vi "FlexMag - 23-03-2023.vi"() -> ()   [LabVIEW 2018] (continued)
              }
              frame #16 {
                n12360 = local read "ch4-3 transfer"() -> (w17570:bool)
                n12361 = case shown="True" w17570 {
                  frame False {
                  }
                  frame True {
                    n12362 = local read "ABORT"() -> (w17571:bool)
                    n12363 = case shown="False" w17571 {
                      frame False {
                        n12364 = local write "trns 4-3 led 7"(TRUE ("trns 1-2 led 1")) -> ()
                        n12365 = Wait (ms)(milliseconds to wait=u32 100) -> ()  [unwired: 1 out]
                      }
                      frame True {
                      }
                    }
                  }
                }
              }
              frame #17 {
                n12366 = local read "ch4-3 transfer"() -> (w17574:bool)
                n12367 = case shown="True" w17574 {
                  frame False {
                  }
                  frame True {
                    n12368 = local read "ABORT"() -> (w17575:bool)
                    n12369 = case shown="False" w17575 {
                      frame False {
                        n12370 = disable-structure shown="Enabled" {
                          frame Disabled {
                            n12371 = while {
                              i -> [w17580]
                              stop <- w17581 stop-if-true
                              n12372 = Greater Or Equal?(x=w17580, y=100) -> (x >= y?=w17578:bool)
                              n12373 = case shown="True" w17578 {
                                frame False {
                                }
                                frame True {
                                n12374 = local write "Warning Message"("Transfer process canceled!\nRight Slow Sensor problem" ("Warning Message")) -> ()
                                n12375 = local write "trns error"(TRUE ("TRNS error")) -> ()
                                }
                              }
                              n12376 = local read "Cnt_Right_Slow DI"() -> (w17576:bool)
                              n12377 = case shown="True" w17576 {
                                tunnel: [TRUE ("CH1_Trns_BP_Left_DO") FALSE ("CH1_Trns_BP_Left_DO")] -> w17577
                                frame False {
                                }
                                frame True {
                                n12378 = Wait Until Next ms Multiple(millisecond multiple=u32 200) -> ()  [unwired: 1 out]
                                n12379 = local write "Cnt_Right_Slow DO"(FALSE ("CH1_Trns_BP_Left_DO")) -> ()
                                }
                              }
                              n12380 = local read "ch4-3 transfer"() -> (w17584:bool)
                              n12381 = local read "ABORT"() -> (w17583:bool)
                              n12382 = Not(x=w17584) -> (.not. x?=w17582:bool)
                              n12383 = Compound Arithmetic op=OR(w17577, w17583, w17582) -> (w17581:bool)
                            }
                          }
                          frame Enabled {
                          }
                        }
                      }
                      frame True {
                      }
                    }
                  }
                }
              }
              frame #18 {
                n12384 = local read "ch4-3 transfer"() -> (w17591:bool)
                n12385 = case shown="True" w17591 {
                  frame False {
                  }
                  frame True {
                    n12386 = local read "ABORT"() -> (w17592:bool)
                    n12387 = case shown="False" w17592 {
                      frame False {
                        n12388 = local write "trns 4-3 led 8"(TRUE ("trns 1-2 led 1")) -> ()
                        n12389 = Wait (ms)(milliseconds to wait=u32 100) -> ()  [unwired: 1 out]
                      }
                      frame True {
                      }
                    }
                  }
                }
              }
              frame #19 {
                n12390 = local read "ch4-3 transfer"() -> (w17595:bool)
                n12391 = case shown="True" w17595 {
                  frame False {
                  }
                  frame True {
                    n12392 = local read "ABORT"() -> (w17596:bool)
                    n12393 = case shown="False" w17596 {
                      frame False {
                        n12394 = disable-structure shown="Enabled" {
                          frame Disabled {
                            n12395 = while {
                              i -> [w17601]
                              stop <- w17602 stop-if-true
                              n12396 = Greater Or Equal?(x=w17601, y=100) -> (x >= y?=w17599:bool)
                              n12397 = case shown="True" w17599 {
                                frame False {
                                }
                                frame True {
                                n12398 = local write "Warning Message"("Transfer process canceled!\nRight Limit Sensor problem" ("Warning Message")) -> ()
                                n12399 = local write "trns error"(TRUE ("TRNS error")) -> ()
                                }
                              }
                              n12400 = local read "Cnt_Right_Limit DI"() -> (w17597:bool)
                              n12401 = case shown="True" w17597 {
                                tunnel: [TRUE ("CH1_Trns_BP_Left_DO") FALSE ("CH1_Trns_BP_Left_DO")] -> w17598
                                frame False {
                                }
                                frame True {
                                n12402 = Wait Until Next ms Multiple(millisecond multiple=u32 200) -> ()  [unwired: 1 out]
                                n12403 = local write "Cnt_Right_Limit DO"(FALSE ("CH1_Trns_BP_Left_DO")) -> ()
                                }
                              }
                              n12404 = local read "ch4-3 transfer"() -> (w17605:bool)
                              n12405 = local read "ABORT"() -> (w17604:bool)
                              n12406 = Not(x=w17605) -> (.not. x?=w17603:bool)
                              n12407 = Compound Arithmetic op=OR(w17598, w17604, w17603) -> (w17602:bool)
                            }
                          }
                          frame Enabled {
                            w17613 = TRUE
                            w17614 = FALSE
                            n12408 = local write "CH3_Right_Limit_DO"(w17614) -> ()
                            n12409 = local write "CH3_Right_Slow_DO"(w17614) -> ()
                            n12410 = local write "CH3_Left_Slow_DO"(w17613) -> ()
                            n12411 = local write "CH3_Left_Limit_DO"(w17613) -> ()
                            n12412 = Wait (ms)(milliseconds to wait=u32 2000) -> ()  [unwired: 1 out]
                          }
                        }
                      }
                      frame True {
                      }
                    }
                  }
                }
              }
              frame #20 {
                n12413 = local read "ch4-3 transfer"() -> (w17615:bool)
                n12414 = case shown="True" w17615 {
                  frame False {
                  }
                  frame True {
                    n12415 = local read "ABORT"() -> (w17616:bool)
                    n12416 = case shown="False" w17616 {
                      frame False {
                        n12417 = local write "trns 4-3 led 9"(TRUE ("trns 1-2 led 1")) -> ()
                        n12418 = Wait (ms)(milliseconds to wait=u32 100) -> ()  [unwired: 1 out]
                      }
                      frame True {
                      }
                    }
                  }
                }
              }
              frame #21 {
                n12419 = local read "ch4-3 transfer"() -> (w17619:bool)
                n12420 = case shown="True" w17619 {
                  frame False {
                  }
                  frame True {
                    n12421 = local read "ABORT"() -> (w17620:bool)
                    n12422 = case shown="False" w17620 {
                      frame False {
                        n12423 = while {
                          i -> [w17624]
                          stop <- w17625 stop-if-true
                          n12424 = Greater Or Equal?(x=w17624, y=100) -> (x >= y?=w17622:bool)
                          n12425 = case shown="True" w17622 {
                            frame False {
                            }
                            frame True {
                              n12426 = local write "Warning Message"("Transfer process canceled!\nLeft Slow Sensor problem" ("Warning Message")) -> ()
                              n12427 = local write "trns error"(TRUE ("TRNS error")) -> ()
                            }
                          }
                          n12428 = disable-structure shown="Enabled" {
                            disable-tunnel: [w17630 w17635] -> w17621
                            frame Disabled {
                              n12429 = local read "Cnt_Left_Slow DI"() -> (w17629:bool)
                              n12430 = case shown="False" w17629 {
                                tunnel: [FALSE ("CH1_Trns_BP_Left_DO") TRUE ("CH1_Trns_BP_Left_DO")] -> w17630
                                frame False {
                                n12431 = Wait Until Next ms Multiple(millisecond multiple=u32 200) -> ()  [unwired: 1 out]
                                n12432 = local write "Cnt_Left_Slow DO"(TRUE ("CH1_Trns_BP_Left_DO")) -> ()
                                }
                                frame True {
                                }
                              }
                            }
                            frame Enabled {
                              n12433 = local read "CH4_Left_Slow_DI"() -> (w17636:bool)
                              n12434 = case shown="True" w17636 {
                                tunnel: [TRUE FALSE] -> w17635
                                frame False {
                                }
                                frame True {
                                n12435 = Wait Until Next ms Multiple(millisecond multiple=u32 200) -> ()  [unwired: 1 out]
                                n12436 = local write "CH4_Left_Slow_DO"(TRUE ("CH2_Right_Limit_DO")) -> ()
                                }
                              }
                            }
                          }
                          n12437 = local read "ch4-3 transfer"() -> (w17628:bool)
                          n12438 = local read "ABORT"() -> (w17627:bool)
                          n12439 = Not(x=w17628) -> (.not. x?=w17626:bool)
                          n12440 = Compound Arithmetic op=OR(w17621, w17627, w17626) -> (w17625:bool)
                        }
                      }
                      frame True {
                      }
                    }
                  }
                }
              }
              frame #22 {
                n12441 = local read "ch4-3 transfer"() -> (w17643:bool)
                n12442 = case shown="True" w17643 {
                  frame False {
                  }
                  frame True {
                    n12443 = local read "ABORT"() -> (w17644:bool)
                    n12444 = case shown="False" w17644 {
                      frame False {
                        n12445 = local write "trns 4-3 led 10"(TRUE ("trns 1-2 led 1")) -> ()
                        n12446 = Wait (ms)(milliseconds to wait=u32 100) -> ()  [unwired: 1 out]
                      }
                      frame True {
                      }
                    }
                  }
                }
              }
              frame #23 {
                n12447 = local read "ch4-3 transfer"() -> (w17647:bool)
                n12448 = case shown="True" w17647 {
                  frame False {
                  }
                  frame True {
                    n12449 = local read "ABORT"() -> (w17648:bool)
                    n12450 = case shown="False" w17648 {
                      frame False {
                        n12451 = while {
                          i -> [w17652]
                          stop <- w17653 stop-if-true
                          n12452 = Greater Or Equal?(x=w17652, y=100) -> (x >= y?=w17650:bool)
                          n12453 = case shown="True" w17650 {
                            frame False {
                            }
                            frame True {
                              n12454 = local write "Warning Message"("Transfer process canceled!\nLeft Limit Sensor problem" ("Warning Message")) -> ()
                              n12455 = local write "trns error"(TRUE ("TRNS error")) -> ()
                            }
                          }
                          n12456 = disable-structure shown="Enabled" {
                            disable-tunnel: [w17658 w17663] -> w17649
                            frame Disabled {
                              n12457 = local read "Cnt_Left_Limit DI"() -> (w17657:bool)
                              n12458 = case shown="False" w17657 {
                                tunnel: [FALSE ("CH1_Trns_BP_Left_DO") TRUE ("CH1_Trns_BP_Left_DO")] -> w17658
                                frame False {
                                n12459 = Wait Until Next ms Multiple(millisecond multiple=u32 200) -> ()  [unwired: 1 out]
                                n12460 = local write "Cnt_Left_Limit DO"(TRUE ("CH1_Trns_BP_Left_DO")) -> ()
                                }
                                frame True {
                                }
                              }
                            }
                            frame Enabled {
                              n12461 = local read "CH4_Left_Limit_DI"() -> (w17664:bool)
                              n12462 = case shown="True" w17664 {
                                tunnel: [TRUE FALSE] -> w17663
                                frame False {
                                }
                                frame True {
                                n12463 = Wait Until Next ms Multiple(millisecond multiple=u32 200) -> ()  [unwired: 1 out]
                                n12464 = local write "CH4_Left_Limit_DO"(TRUE ("CH2_Right_Limit_DO")) -> ()
                                }
                              }
                            }
                          }
                          n12465 = local read "ch4-3 transfer"() -> (w17656:bool)
                          n12466 = local read "ABORT"() -> (w17655:bool)
                          n12467 = Not(x=w17656) -> (.not. x?=w17654:bool)
                          n12468 = Compound Arithmetic op=OR(w17649, w17655, w17654) -> (w17653:bool)
                        }
                      }
                      frame True {
                      }
                    }
                  }
                }
              }
              frame #24 {
                n12469 = local read "ch4-3 transfer"() -> (w17671:bool)
                n12470 = case shown="True" w17671 {
                  frame False {
                  }
                  frame True {
                    n12471 = local read "ABORT"() -> (w17672:bool)
                    n12472 = case shown="False" w17672 {
                      frame False {
                        n12473 = local write "trns 4-3 led 11"(TRUE ("trns 1-2 led 1")) -> ()
                        n12474 = Wait (ms)(milliseconds to wait=u32 100) -> ()  [unwired: 1 out]
                      }
                      frame True {
                      }
                    }
                  }
                }
              }
              frame #25 {
                n12475 = local read "ch4-3 transfer"() -> (w17675:bool)
                n12476 = case shown="True" w17675 {
                  frame False {
                  }
                  frame True {
                    n12477 = local read "ABORT"() -> (w17676:bool)
                    n12478 = case shown="False" w17676 {
                      frame False {
                        n12479 = while {
                          i -> [w17681]
                          stop <- w17682 stop-if-true
                          n12480 = Greater Or Equal?(x=w17681, y=100) -> (x >= y?=w17679:bool)
                          n12481 = case shown="True" w17679 {
                            frame False {
                            }
                            frame True {
                              n12482 = local write "Warning Message"("Transfer process canceled!\nCassette Servo Direction problem" ("Warning Message")) -> ()
                              n12483 = local write "trns error"(TRUE ("TRNS error")) -> ()
                            }
                          }
                          n12484 = local read "Casette_Servo_Left_Direction DI"() -> (w17677:bool)
                          n12485 = case shown="True" w17677 {
                            tunnel: [TRUE ("CH1_Trns_BP_Left_DO") FALSE ("CH1_Trns_BP_Left_DO")] -> w17678
                            frame False {
                            }
                            frame True {
                              n12486 = local write "Casette_Servo_Left_Direction DO"(FALSE ("CH1_Trns_BP_Left_DO")) -> ()
                              n12487 = Wait Until Next ms Multiple(millisecond multiple=u32 200) -> ()  [unwired: 1 out]
                            }
                          }
                          n12488 = local read "ch4-3 transfer"() -> (w17685:bool)
                          n12489 = local read "ABORT"() -> (w17684:bool)
                          n12490 = Not(x=w17685) -> (.not. x?=w17683:bool)
                          n12491 = Compound Arithmetic op=OR(w17678, w17684, w17683) -> (w17682:bool)
                        }
                      }
                      frame True {
                      }
                    }
                  }
                }
              }
              frame #26 {
                n12492 = local read "ch4-3 transfer"() -> (w17692:bool)
                n12493 = case shown="True" w17692 {
                  frame False {
                  }
                  frame True {
                    n12494 = local read "ABORT"() -> (w17693:bool)
                    n12495 = case shown="False" w17693 {
                      frame False {
                        n12496 = local write "trns 4-3 led 12"(TRUE ("trns 1-2 led 1")) -> ()
                        n12497 = Wait (ms)(milliseconds to wait=u32 100) -> ()  [unwired: 1 out]
                      }
                      frame True {
                      }
                    }
                  }
                }
              }
              frame #27 {
                n12498 = local read "ch4-3 transfer"() -> (w17696:bool)
                n12499 = case shown="True" w17696 {
                  frame False {
                  }
                  frame True {
                    n12500 = local read "ABORT"() -> (w17697:bool)
                    n12501 = case shown="False" w17697 {
                      frame False {
                        n12502 = stacked-sequence {
                          frame #0 {
                            n12503 = local read "Cst_Speed_High"() -> (w17698:dbl)
                            n12504 = Wait (ms)(milliseconds to wait=u32 100) -> ()  [unwired: 1 out]
                            n12505 = local write "Cassette_Servo_Speed AO"(w17698) -> ()
                          }
                          frame #1 {
                            n12506 = Wait (ms)(milliseconds to wait=u32 200) -> ()  [unwired: 1 out]
                          }
                          frame #2 {
                            n12507 = local write "Cassette_Servo_Speed Set"(TRUE ("Cassette_Servo_Speed Set")) -> ()
                          }
                          frame #3 {
                            n12508 = Wait (ms)(milliseconds to wait=u32 300) -> ()  [unwired: 1 out]
                          }
                        }
                      }
                      frame True {
                      }
                    }
                  }
                }
              }
              frame #28 {
                n12509 = local read "ch4-3 transfer"() -> (w17703:bool)
                n12510 = case shown="True" w17703 {
                  frame False {
                  }
                  frame True {
                    n12511 = local read "ABORT"() -> (w17704:bool)
                    n12512 = case shown="False" w17704 {
                      frame False {
                        n12513 = local write "trns 4-3 led 13"(TRUE ("trns 1-2 led 1")) -> ()
                        n12514 = Wait (ms)(milliseconds to wait=u32 100) -> ()  [unwired: 1 out]
                      }
                      frame True {
                      }
                    }
                  }
                }
              }
              frame #29 {
                n12515 = local read "ch4-3 transfer"() -> (w17707:bool)
                n12516 = case shown="True" w17707 {
                  frame False {
                  }
                  frame True {
                    n12517 = local read "ABORT"() -> (w17708:bool)
                    n12518 = case shown="False" w17708 {
                      frame False {
                        n12519 = while {
                          i -> [w17713]
                          stop <- w17714 stop-if-true
                          n12520 = Greater Or Equal?(x=w17713, y=100) -> (x >= y?=w17711:bool)
                          n12521 = case shown="True" w17711 {
                            frame False {
                            }
                            frame True {
                              n12522 = local write "Warning Message"("Transfer process canceled!\nCassette Servo Start problem" ("Warning Message")) -> ()
                              n12523 = local write "trns error"(TRUE ("TRNS error")) -> ()
                            }
                          }
                          n12524 = local read "Casette_Servo_Start/Stop DI"() -> (w17709:bool)
                          n12525 = case shown="False" w17709 {
                            tunnel: [FALSE ("CH1_Trns_BP_Left_DO") TRUE ("CH1_Trns_BP_Left_DO")] -> w17710
                            frame False {
                              n12526 = local write "Casette_Servo_Start/Stop DO"(TRUE ("CH1_Trns_BP_Left_DO")) -> ()
                              n12527 = Wait Until Next ms Multiple(millisecond multiple=u32 200) -> ()  [unwired: 1 out]
                            }
                            frame True {
                            }
                          }
                          n12528 = local read "ch4-3 transfer"() -> (w17717:bool)
                          n12529 = local read "ABORT"() -> (w17716:bool)
                          n12530 = Not(x=w17717) -> (.not. x?=w17715:bool)
                          n12531 = Compound Arithmetic op=OR(w17710, w17716, w17715) -> (w17714:bool)
                        }
                      }
                      frame True {
                      }
                    }
                  }
                }
              }
              frame #30 {
                n12532 = local read "ch4-3 transfer"() -> (w17724:bool)
                n12533 = case shown="True" w17724 {
                  frame False {
                  }
                  frame True {
                    n12534 = local read "ABORT"() -> (w17725:bool)
                    n12535 = case shown="False" w17725 {
                      frame False {
                        n12536 = local write "trns 4-3 led 14"(TRUE ("trns 1-2 led 1")) -> ()
                        n12537 = Wait (ms)(milliseconds to wait=u32 100) -> ()  [unwired: 1 out]
                      }
                      frame True {
                      }
                    }
                  }
                }
              }
              frame #31 {
                n12538 = local read "ch4-3 transfer"() -> (w17728:bool)
                n12539 = case shown="True" w17728 {
                  frame False {
                  }
                  frame True {
                    n12540 = local read "ABORT"() -> (w17729:bool)
                    n12541 = case shown="False" w17729 {
                      frame False {
                        n12542 = stacked-sequence {
                          frame #0 {
                            n12543 = while {
                              i -> [w17734]
                              stop <- w17735 stop-if-true
                              n12544 = Greater Or Equal?(x=w17734, y=1500) -> (x >= y?=w17732:bool)
                              n12545 = case shown="True" w17732 {
                                frame False {
                                }
                                frame True {
                                n12546 = local write "Warning Message"("Transfer process canceled!\nCH3 Right Slow Sensor problem" ("Warning Message")) -> ()
                                n12547 = local write "trns error"(TRUE ("TRNS error")) -> ()
                                }
                              }
                              n12548 = local read "CH3_Right_Slow_DI"() -> (w17730:bool)
                              n12549 = case shown="True" w17730 {
                                tunnel: [FALSE ("CH1_Trns_BP_Left_DO") TRUE ("CH1_Trns_BP_Left_DO")] -> w17731
                                frame False {
                                n12550 = Wait Until Next ms Multiple(millisecond multiple=u32 200) -> ()  [unwired: 1 out]
                                }
                                frame True {
                                }
                              }
                              n12551 = local read "ch4-3 transfer"() -> (w17738:bool)
                              n12552 = local read "ABORT"() -> (w17737:bool)
                              n12553 = Not(x=w17738) -> (.not. x?=w17736:bool)
                              n12554 = Compound Arithmetic op=OR(w17731, w17737, w17736) -> (w17735:bool)
                            }
                          }
                          frame #1 {
                            n12555 = flat-sequence {
                              frame #0 {
                                n12556 = local read "Cst_Speed_Low"() -> (w17744:dbl)
                                n12557 = local write "Cassette_Servo_Speed AO"(w17744) -> ()
                                n12558 = Wait (ms)(milliseconds to wait=u32 100) -> ()  [unwired: 1 out]
                              }
                              frame #1 {
                                n12559 = local write "Cassette_Servo_Speed Set"(TRUE ("Cassette_Servo_Speed Set")) -> ()
                              }
                              frame #2 {
                                n12560 = Wait (ms)(milliseconds to wait=u32 100) -> ()  [unwired: 1 out]
                              }
                            }
                          }
                          frame #2 {
                            n12561 = while {
                              i -> [w17751]
                              stop <- w17752 stop-if-true
                              n12562 = Greater Or Equal?(x=w17751, y=100) -> (x >= y?=w17749:bool)
                              n12563 = case shown="True" w17749 {
                                frame False {
                                }
                                frame True {
                                n12564 = local write "Warning Message"("Transfer process canceled!\nRight Slow Sensor problem" ("Warning Message")) -> ()
                                n12565 = local write "trns error"(TRUE ("TRNS error")) -> ()
                                }
                              }
                              n12566 = disable-structure shown="Enabled" {
                                disable-tunnel: [w17757 w17762] -> w17748
                                frame Disabled {
                                n12567 = local read "Cnt_Right_Slow DI"() -> (w17756:bool)
                                n12568 = case shown="False" w17756 {
                                tunnel: [FALSE ("CH1_Trns_BP_Left_DO") TRUE ("CH1_Trns_BP_Left_DO")] -> w17757
                                frame False {
                                n12569 = Wait Until Next ms Multiple(millisecond multiple=u32 200) -> ()  [unwired: 1 out]
                                n12570 = local write "Cnt_Right_Slow DO"(TRUE ("TRNS error")) -> ()
                                }
                                frame True {
                                }
                                }
                                }
                                frame Enabled {
                                n12571 = local read "CH3_Right_Slow_DI"() -> (w17763:bool)
                                n12572 = case shown="True" w17763 {
                                tunnel: [TRUE FALSE] -> w17762
                                frame False {
                                }
                                frame True {
                                n12573 = Wait Until Next ms Multiple(millisecond multiple=u32 200) -> ()  [unwired: 1 out]
                                n12574 = local write "CH3_Right_Slow_DO"(TRUE ("CH2_Right_Limit_DO")) -> ()
                                }
                                }
                                }
                              }
                              n12575 = local read "ch4-3 transfer"() -> (w17755:bool)
                              n12576 = local read "ABORT"() -> (w17754:bool)
                              n12577 = Not(x=w17755) -> (.not. x?=w17753:bool)
                              n12578 = Compound Arithmetic op=OR(w17748, w17754, w17753) -> (w17752:bool)
                            }
                          }
                        }
                      }
                      frame True {
                      }
                    }
                  }
                }
              }
              frame #32 {
                n12579 = local read "ch4-3 transfer"() -> (w17770:bool)
                n12580 = case shown="True" w17770 {
                  frame False {
                  }
                  frame True {
                    n12581 = local read "ABORT"() -> (w17771:bool)
                    n12582 = case shown="False" w17771 {
                      frame False {
                        n12583 = local write "trns 4-3 led 15"(TRUE ("trns 1-2 led 1")) -> ()
                        n12584 = Wait (ms)(milliseconds to wait=u32 100) -> ()  [unwired: 1 out]
                      }
                      frame True {
                      }
                    }
                  }
                }
              }
              frame #33 {
                n12585 = local read "ch4-3 transfer"() -> (w17774:bool)
                n12586 = case shown="True" w17774 {
                  frame False {
                  }
                  frame True {
                    n12587 = local read "ABORT"() -> (w17775:bool)
                    n12588 = case shown="False" w17775 {
                      frame False {
                        n12589 = stacked-sequence {
                          frame #0 {
                            n12590 = while {
                              i -> [w17780]
                              stop <- w17781 stop-if-true
                              n12591 = Greater Or Equal?(x=w17780, y=600) -> (x >= y?=w17778:bool)
                              n12592 = case shown="True" w17778 {
                                frame False {
                                }
                                frame True {
                                n12593 = local write "Warning Message"("Transfer process canceled!\nCH3 Right Limit Sensor problem" ("Warning Message")) -> ()
                                n12594 = local write "trns error"(TRUE ("TRNS error")) -> ()
                                }
                              }
                              n12595 = local read "CH3_Right_Limit_DI"() -> (w17776:bool)
                              n12596 = case shown="True" w17776 {
                                tunnel: [FALSE ("CH1_Trns_BP_Left_DO") TRUE ("CH1_Trns_BP_Left_DO")] -> w17777
                                frame False {
                                n12597 = Wait Until Next ms Multiple(millisecond multiple=u32 200) -> ()  [unwired: 1 out]
                                }
                                frame True {
                                }
                              }
                              n12598 = local read "ch4-3 transfer"() -> (w17784:bool)
                              n12599 = local read "ABORT"() -> (w17783:bool)
                              n12600 = Not(x=w17784) -> (.not. x?=w17782:bool)
                              n12601 = Compound Arithmetic op=OR(w17777, w17783, w17782) -> (w17781:bool)
                            }
                          }
                          frame #1 {
                            n12602 = while {
                              i -> [w17794]
                              stop <- w17795 stop-if-true
                              n12603 = Greater Or Equal?(x=w17794, y=100) -> (x >= y?=w17792:bool)
                              n12604 = case shown="True" w17792 {
                                frame False {
                                }
                                frame True {
                                n12605 = local write "Warning Message"("Transfer process canceled!\nCassette Servo couldn't be stopped" ("Warning Message")) -> ()
                                n12606 = local write "trns error"(TRUE ("TRNS error")) -> ()
                                }
                              }
                              n12607 = local read "Casette_Servo_Start/Stop DI"() -> (w17790:bool)
                              n12608 = case shown="True" w17790 {
                                tunnel: [TRUE ("CH1_Trns_BP_Left_DO") FALSE ("CH1_Trns_BP_Left_DO")] -> w17791
                                frame False {
                                }
                                frame True {
                                n12609 = Wait Until Next ms Multiple(millisecond multiple=u32 200) -> ()  [unwired: 1 out]
                                n12610 = local write "Casette_Servo_Start/Stop DO"(FALSE ("TRNS error")) -> ()
                                }
                              }
                              n12611 = local read "ch4-3 transfer"() -> (w17798:bool)
                              n12612 = local read "ABORT"() -> (w17797:bool)
                              n12613 = Not(x=w17798) -> (.not. x?=w17796:bool)
                              n12614 = Compound Arithmetic op=OR(w17791, w17797, w17796) -> (w17795:bool)
                            }
                          }
                          frame #2 {
                            n12615 = flat-sequence {
                              frame #0 {
                                n12616 = local write "Cassette_Servo_Speed AO"(0.0 ("Cassette_Servo_Speed AO")) -> ()
                                n12617 = Wait (ms)(milliseconds to wait=u32 100) -> ()  [unwired: 1 out]
                              }
                              frame #1 {
                                n12618 = local write "Cassette_Servo_Speed Set"(TRUE ("Cassette_Servo_Speed Set")) -> ()
                              }
                            }
                          }
                        }
                      }
                      frame True {
                      }
                    }
                  }
                }
              }
              frame #34 {
                n12619 = local read "ch4-3 transfer"() -> (w17808:bool)
                n12620 = case shown="True" w17808 {
                  frame False {
                  }
                  frame True {
                    n12621 = local read "ABORT"() -> (w17809:bool)
                    n12622 = case shown="False" w17809 {
                      frame False {
                        n12623 = local write "trns 4-3 led 16"(TRUE ("trns 1-2 led 1")) -> ()
                        n12624 = Wait (ms)(milliseconds to wait=u32 100) -> ()  [unwired: 1 out]
                      }
                      frame True {
                      }
                    }
                  }
                }
              }
              frame #35 {
                n12625 = local read "ch4-3 transfer"() -> (w17812:bool)
                n12626 = case shown="True" w17812 {
                  frame False {
                  }
                  frame True {
                    n12627 = local read "ABORT"() -> (w17813:bool)
                    n12628 = case shown="False" w17813 {
                      frame False {
                        n12629 = local read "target chamber"() -> (w17814:dbl)
                        n12630 = Equal?(x=w17814, y=3.0) -> (x = y?=w17815:bool)
                        n12631 = case shown="True" w17815 {
                          frame False {
                          }
                          frame True {
                            n12632 = while {
                              i -> [w17821]
                              stop <- w17822 stop-if-true
                              n12633 = Greater Or Equal?(x=w17821, y=100) -> (x >= y?=w17819:bool)
                              n12634 = case shown="True" w17819 {
                                frame False {
                                }
                                frame True {
                                n12635 = local write "Warning Message"("Transfer process canceled!\nCH3 Cassette Fix couldn't reached  to down position" ("Warning Message")) -> ()
                                n12636 = local write "trns error"(TRUE ("TRNS error")) -> ()
                                }
                              }
                              n12637 = local read "CH3_Cst_Fix_Down_DI"() -> (w17817:bool)
                              n12638 = case shown="False" w17817 {
                                tunnel: [FALSE ("CH1_Trns_BP_Left_DO") TRUE ("CH1_Trns_BP_Left_DO")] -> w17818
                                frame False {
                                n12639 = Wait Until Next ms Multiple(millisecond multiple=u32 200) -> ()  [unwired: 1 out]
                                n12640 = local write "CH3_Cst_Fix_DO"(TRUE ("TRNS error")) -> ()
                                }
                                frame True {
                                }
                              }
                              n12641 = local read "ch4-3 transfer"() -> (w17825:bool)
                              n12642 = local read "ABORT"() -> (w17824:bool)
                              n12643 = Not(x=w17825) -> (.not. x?=w17823:bool)
                              n12644 = Compound Arithmetic op=OR(w17818, w17824, w17823) -> (w17822:bool)
                            }
                          }
                        }
                      }
                      frame True {
                      }
                    }
                  }
                }
              }
              frame #36 {
                n12645 = local read "ch4-3 transfer"() -> (w17832:bool)
                n12646 = case shown="True" w17832 {
                  frame False {
                  }
                  frame True {
                    n12647 = local read "ABORT"() -> (w17833:bool)
                    n12648 = case shown="False" w17833 {
                      frame False {
                        n12649 = local write "trns 4-3 led 17"(TRUE ("trns 1-2 led 1")) -> ()
                        n12650 = Wait (ms)(milliseconds to wait=u32 100) -> ()  [unwired: 1 out]
                      }
                      frame True {
                      }
                    }
                  }
                }
              }
              frame #37 {
                n12651 = local read "ch4-3 transfer"() -> (w17836:bool)
                n12652 = case shown="True" w17836 {
                  frame False {
                  }
                  frame True {
                    n12653 = local read "ABORT"() -> (w17837:bool)
                    n12654 = case shown="False" w17837 {
                      frame False {
                        n12655 = while {
                          i -> [w17842]
                          stop <- w17843 stop-if-true
                          n12656 = Greater Or Equal?(x=w17842, y=100) -> (x >= y?=w17840:bool)
                          n12657 = case shown="True" w17840 {
                            frame False {
                            }
                            frame True {
                              n12658 = local write "Warning Message"("Transfer process canceled!\nCH3 Trns Bp Left coulnt't be closed" ("Warning Message")) -> ()
                              n12659 = local write "trns error"(TRUE ("TRNS error")) -> ()
                            }
                          }
                          n12660 = local read "CH3_Trns_BP_Left_DI"() -> (w17838:bool)
                          n12661 = case shown="True" w17838 {
                            tunnel: [TRUE ("CH1_Trns_BP_Left_DO") FALSE ("CH1_Trns_BP_Left_DO")] -> w17839
                            frame False {
                            }
                            frame True {
                              n12662 = Wait Until Next ms Multiple(millisecond multiple=u32 200) -> ()  [unwired: 1 out]
                              n12663 = local write "CH3_Trns_BP_Left_DO"(FALSE ("TRNS error")) -> ()
                            }
                          }
                          n12664 = local read "ch4-3 transfer"() -> (w17846:bool)
                          n12665 = local read "ABORT"() -> (w17845:bool)
                          n12666 = Not(x=w17846) -> (.not. x?=w17844:bool)
                          n12667 = Compound Arithmetic op=OR(w17839, w17845, w17844) -> (w17843:bool)
                        }
                      }
                      frame True {
                      }
                    }
                  }
                }
              }
              frame #38 {
                n12668 = local read "ch4-3 transfer"() -> (w17853:bool)
                n12669 = case shown="True" w17853 {
                  frame False {
                  }
                  frame True {
                    n12670 = local read "ABORT"() -> (w17854:bool)
                    n12671 = case shown="False" w17854 {
                      frame False {
                        n12672 = local write "trns 4-3 led 18"(TRUE ("trns 1-2 led 1")) -> ()
                        n12673 = Wait (ms)(milliseconds to wait=u32 100) -> ()  [unwired: 1 out]
                      }
                      frame True {
                      }
                    }
                  }
                }
              }
              frame #39 {
                n12674 = local read "ch4-3 transfer"() -> (w17857:bool)
                n12675 = case shown="True" w17857 {
                  frame False {
                  }
                  frame True {
                    n12676 = local read "ABORT"() -> (w17858:bool)
                    n12677 = case shown="False" w17858 {
                      frame False {
                        n12678 = while {
                          i -> [w17863]
                          stop <- w17864 stop-if-true
                          n12679 = Greater Or Equal?(x=w17863, y=100) -> (x >= y?=w17861:bool)
                          n12680 = case shown="True" w17861 {
                            frame False {
                            }
                            frame True {
                              n12681 = local write "Warning Message"("Transfer process canceled!\nCH4 Trns Bp Right coulnt't be closed" ("Warning Message")) -> ()
                              n12682 = local write "trns error"(TRUE ("TRNS error")) -> ()
                            }
                          }
                          n12683 = local read "CH4_Trns_BP_Right_DI"() -> (w17859:bool)
                          n12684 = case shown="True" w17859 {
                            tunnel: [TRUE ("CH1_Trns_BP_Left_DO") FALSE ("CH1_Trns_BP_Left_DO")] -> w17860
                            frame False {
                            }
                            frame True {
                              n12685 = local write "CH4_Trns_BP_Right_DO"(FALSE ("TRNS error")) -> ()
                              n12686 = Wait Until Next ms Multiple(millisecond multiple=u32 200) -> ()  [unwired: 1 out]
                            }
                          }
                          n12687 = local read "ch4-3 transfer"() -> (w17867:bool)
                          n12688 = local read "ABORT"() -> (w17866:bool)
                          n12689 = Not(x=w17867) -> (.not. x?=w17865:bool)
                          n12690 = Compound Arithmetic op=OR(w17860, w17866, w17865) -> (w17864:bool)
                        }
                      }
                      frame True {
                      }
                    }
                  }
                }
              }
              frame #40 {
                n12691 = local read "ch4-3 transfer"() -> (w17874:bool)
                n12692 = case shown="True" w17874 {
                  frame False {
                  }
                  frame True {
                    n12693 = local read "ABORT"() -> (w17875:bool)
                    n12694 = case shown="False" w17875 {
                      frame False {
                        n12695 = local write "trns 4-3 led 19"(TRUE ("trns 1-2 led 1")) -> ()
                        n12696 = Wait (ms)(milliseconds to wait=u32 100) -> ()  [unwired: 1 out]
                      }
                      frame True {
                      }
                    }
                  }
                }
              }
              frame #41 {
                n12697 = local read "ch4-3 transfer"() -> (w17878:bool)
                n12698 = case shown="True" w17878 {
                  frame False {
                  }
                  frame True {
                    n12699 = local read "ABORT"() -> (w17879:bool)
                    n12700 = case shown="False" w17879 {
                      frame False {
                        n12701 = stacked-sequence {
                          frame #0 {
                            n12702 = local read "ch4-3 transfer"() -> (w17880:bool)
                            n12703 = case shown="True" w17880 {
                              frame False {
                              }
                              frame True {
                                n12704 = local write "CH3_Trns_GV_Open_DO"(FALSE ("trns clear")) -> ()
                              }
                            }
                          }
                          frame #1 {
                            n12705 = while {
                              i -> [w17886]
                              stop <- w17887 stop-if-true
                              n12706 = Greater Or Equal?(x=w17886, y=600) -> (x >= y?=w17884:bool)
                              n12707 = case shown="True" w17884 {
                                frame False {
                                }
                                frame True {
                                n12708 = local write "Warning Message"("Transfer process canceled!\nCH3-CH4 Trns GV couldn't be closed" ("Warning Message")) -> ()
                                n12709 = local write "trns error"(TRUE ("TRNS error")) -> ()
                                }
                              }
                              n12710 = local read "CH3_Trns_Gv_Close_DI"() -> (w17882:bool)
                              n12711 = case shown="False" w17882 {
                                tunnel: [FALSE ("CH1_Trns_BP_Left_DO") TRUE ("CH1_Trns_BP_Left_DO")] -> w17883
                                frame False {
                                n12712 = local write "CH3_Trns_GV_Close_DO"(TRUE ("TRNS error")) -> ()
                                n12713 = Wait Until Next ms Multiple(millisecond multiple=u32 200) -> ()  [unwired: 1 out]
                                }
                                frame True {
                                }
                              }
                              n12714 = local read "ch4-3 transfer"() -> (w17890:bool)
                              n12715 = local read "ABORT"() -> (w17889:bool)
                              n12716 = Not(x=w17890) -> (.not. x?=w17888:bool)
                              n12717 = Compound Arithmetic op=OR(w17883, w17889, w17888) -> (w17887:bool)
                            }
                          }
                        }
                      }
                      frame True {
                      }
                    }
                  }
                }
              }
              frame #42 {
                n12718 = local read "ch4-3 transfer"() -> (w17897:bool)
                n12719 = case shown="True" w17897 {
                  frame False {
                  }
                  frame True {
                    n12720 = local read "ABORT"() -> (w17898:bool)
                    n12721 = case shown="False" w17898 {
                      frame False {
                        n12722 = local write "trns 4-3 led 20"(TRUE ("trns 1-2 led 1")) -> ()
                        n12723 = Wait (ms)(milliseconds to wait=u32 100) -> ()  [unwired: 1 out]
                      }
                      frame True {
                      }
                    }
                  }
                }
              }
              frame #43 {
                n12724 = local read "ch4-3 transfer"() -> (w17901:bool)
                n12725 = case shown="True" w17901 {
                  frame False {
                  }
                  frame True {
                    n12726 = local read "ABORT"() -> (w17902:bool)
                    n12727 = case shown="False" w17902 {
                      frame False {
                        n12728 = local read "target chamber"() -> (w17903:dbl)
                        n12729 = Equal?(x=w17903, y=3.0) -> (x = y?=w17904:bool)
                        n12730 = case shown="True" w17904 {
                          frame False {
                          }
                          frame True {
                            n12731 = stacked-sequence {
                              frame #0 {
                                n12732 = local read "ch4-3 transfer"() -> (w17906:bool)
                                n12733 = case shown="True" w17906 {
                                frame False {
                                }
                                frame True {
                                n12734 = local write "CH3_PetCool_Up_DO"(FALSE ("trns clear")) -> ()
                                }
                                }
                              }
                              frame #1 {
                                n12735 = while {
                                i -> [w17912]
                                stop <- w17913 stop-if-true
                                n12736 = Greater Or Equal?(x=w17912, y=300) -> (x >= y?=w17910:bool)
                                n12737 = case shown="True" w17910 {
                                frame False {
                                }
                                frame True {
                                n12738 = local write "Warning Message"("Transfer process canceled!\nCH3 Petcool couldn't be down" ("Warning Message")) -> ()
                                n12739 = local write "trns error"(TRUE ("TRNS error")) -> ()
                                }
                                }
                                n12740 = local read "CH3_PetCool_Down_DI"() -> (w17908:bool)
                                n12741 = case shown="False" w17908 {
                                tunnel: [FALSE ("CH1_Trns_BP_Left_DO") TRUE ("CH1_Trns_BP_Left_DO")] -> w17909
                                frame False {
                                n12742 = local write "CH3_PetCool_Down_DO"(TRUE ("TRNS error")) -> ()
                                n12743 = Wait Until Next ms Multiple(millisecond multiple=u32 200) -> ()  [unwired: 1 out]
                                }
                                frame True {
                                }
                                }
                                n12744 = local read "ch4-3 transfer"() -> (w17916:bool)
                                n12745 = local read "ABORT"() -> (w17915:bool)
                                n12746 = Not(x=w17916) -> (.not. x?=w17914:bool)
                                n12747 = Compound Arithmetic op=OR(w17909, w17915, w17914) -> (w17913:bool)
                                }
                              }
                            }
                          }
                        }
                      }
                      frame True {
                      }
                    }
                  }
                }
              }
              frame #44 {
                n12748 = local read "ch4-3 transfer"() -> (w17923:bool)
                n12749 = case shown="True" w17923 {
                  frame False {
                  }
                  frame True {
                    n12750 = local read "ABORT"() -> (w17924:bool)
                    n12751 = case shown="False" w17924 {
                      frame False {
                        n12752 = local write "trns 4-3 led 21"(TRUE ("trns 1-2 led 1")) -> ()
                        n12753 = Wait (ms)(milliseconds to wait=u32 100) -> ()  [unwired: 1 out]
                      }
                      frame True {
                      }
                    }
                  }
                }
              }
              frame #45 {
                n12754 = local read "ch4-3 transfer"() -> (w17927:bool)
                n12755 = case shown="True" w17927 {
                  frame False {
                  }
                  frame True {
                    n12756 = local read "ABORT"() -> (w17928:bool)
                    n12757 = case shown="False" w17928 {
                      frame False {
                        n12758 = local read "target chamber"() -> (w17929:dbl)
                        n12759 = Equal?(x=w17929, y=3.0) -> (x = y?=w17930:bool)
                        n12760 = case shown="True" w17930 {
                          frame False {
                          }
                          frame True {
                            n12761 = stacked-sequence {
                              frame #0 {
                                n12762 = local read "ch4-3 transfer"() -> (w17932:bool)
                                n12763 = case shown="True" w17932 {
                                frame False {
                                }
                                frame True {
                                n12764 = local write "CH3_SRV1_Piston_Back_DO"(FALSE ("trns clear")) -> ()
                                }
                                }
                              }
                              frame #1 {
                                n12765 = while {
                                i -> [w17938]
                                stop <- w17939 stop-if-true
                                n12766 = Greater Or Equal?(x=w17938, y=200) -> (x >= y?=w17936:bool)
                                n12767 = case shown="True" w17936 {
                                frame False {
                                }
                                frame True {
                                n12768 = local write "Warning Message"("Transfer process canceled!\nCH3 Servo Piston couldn't be forward" ("Warning Message")) -> ()
                                n12769 = local write "trns error"(TRUE ("TRNS error")) -> ()
                                }
                                }
                                n12770 = local read "CH3_SRV1_Piston_For_DI"() -> (w17934:bool)
                                n12771 = case shown="False" w17934 {
                                tunnel: [FALSE ("CH1_Trns_BP_Left_DO") TRUE ("CH1_Trns_BP_Left_DO")] -> w17935
                                frame False {
                                n12772 = local write "CH3_SRV1_Piston_For_DO"(TRUE ("TRNS error")) -> ()
                                n12773 = Wait Until Next ms Multiple(millisecond multiple=u32 200) -> ()  [unwired: 1 out]
                                }
                                frame True {
                                }
                                }